vi "FlexMag - 23-03-2023.vi"() -> ()   [LabVIEW 2018] (continued)
                          n16002 = local read "abort ch2"() -> (w20214:bool)
                          n16003 = Not(x=w20216) -> (.not. x?=w20215:bool)
                          n16004 = Compound Arithmetic op=OR(w20211, w20214, w20215) -> (w20217:bool)
                        }
                      }
                      frame True {
                      }
                    }
                  }
                }
              }
              frame #6 {
                n16005 = local read "ch2 shutdown alg"() -> (w20224:bool)
                n16006 = case shown="True" w20224 {
                  frame False {
                  }
                  frame True {
                    n16007 = local read "abort ch2"() -> (w20225:bool)
                    n16008 = case shown="False" w20225 {
                      frame False {
                        n16009 = local write "ch2 sd bg bv close led"(TRUE ("ch1 sd cc close led")) -> ()
                        n16010 = Wait (ms)(milliseconds to wait=u32 1000) -> ()  [unwired: 1 out]
                      }
                      frame True {
                      }
                    }
                  }
                }
              }
              frame #7 {
                # "TP stop"
                n16011 = local read "ch2 shutdown alg"() -> (w20228:bool)
                n16012 = case shown="True" w20228 {
                  frame False {
                  }
                  frame True {
                    n16013 = local read "abort ch2"() -> (w20229:bool)
                    n16014 = case shown="False" w20229 {
                      frame False {
                        n16015 = stacked-sequence {
                          frame #0 {
                            n16016 = flat-sequence {
                              frame #0 {
                                n16017 = local write "Tp2 auto stop"(TRUE ("Tp1 auto stop")) -> ()
                                n16018 = Wait (ms)(milliseconds to wait=u32 100) -> ()  [unwired: 1 out]
                              }
                              frame #1 {
                                n16019 = Wait (ms)(milliseconds to wait=u32 5000) -> ()  [unwired: 1 out]
                              }
                              frame #2 {
                                n16020 = local write "Tp2 auto stop"(TRUE ("Tp1 auto stop")) -> ()
                                n16021 = Wait (ms)(milliseconds to wait=u32 100) -> ()  [unwired: 1 out]
                              }
                            }
                          }
                          frame #1 {
                            n16022 = while {
                              i -> [w20246]
                              stop <- w20241 stop-if-true
                              n16023 = Multiply(x=3000 ("y"), y=5) -> (x*y=w20235:i32)
                              n16024 = Greater Or Equal?(x=w20246, y=w20235) -> (x >= y?=w20240:bool)
                              n16025 = case shown="True" w20240 {
                                frame False {
                                }
                                frame True {
                                n16026 = local write "Warning Message"("CH2 ShutDown process  is canceled !\nCH2 TP couldn't be stopped" ("Warning Message")) -> ()
                                n16027 = local write "ch2 shutdown error"(TRUE ("ch1 pumpdown error")) -> ()
                                }
                              }
                              n16028 = local read "ch2 shutdown alg"() -> (w20244:bool)
                              n16029 = local read "ch2_tp_gui"() -> (w20239:bool)
                              n16030 = local read "abort ch2"() -> (w20242:bool)
                              n16031 = Not(x=w20239) -> (.not. x?=w20238:bool)
                              n16032 = Not(x=w20244) -> (.not. x?=w20243:bool)
                              n16033 = Wait Until Next ms Multiple(millisecond multiple=u32 200) -> ()  [unwired: 1 out]
                              n16034 = Compound Arithmetic op=OR(w20238, w20242, w20243) -> (w20241:bool)
                            }
                          }
                        }
                      }
                      frame True {
                      }
                    }
                  }
                }
              }
              frame #8 {
                n16035 = local read "ch2 shutdown alg"() -> (w20249:bool)
                n16036 = case shown="True" w20249 {
                  frame False {
                  }
                  frame True {
                    n16037 = local read "abort ch2"() -> (w20250:bool)
                    n16038 = case shown="False" w20250 {
                      frame False {
                        n16039 = local write "ch2 sd tp stop led"(TRUE ("ch1 sd cc close led")) -> ()
                        n16040 = Wait (ms)(milliseconds to wait=u32 1000) -> ()  [unwired: 1 out]
                      }
                      frame True {
                      }
                    }
                  }
                }
              }
              frame #9 {
                # "tp bv close"
                n16041 = local read "ch2 shutdown alg"() -> (w20253:bool)
                n16042 = case shown="True" w20253 {
                  frame False {
                  }
                  frame True {
                    n16043 = local read "abort ch2"() -> (w20254:bool)
                    n16044 = case shown="False" w20254 {
                      frame False {
                        n16045 = while {
                          i -> [w20259]
                          stop <- w20263 stop-if-true
                          n16046 = Greater?(x=w20259, y=100) -> (0:w20256:bool)
                          n16047 = case shown="True" w20256 {
                            frame False {
                            }
                            frame True {
                              n16048 = local write "Warning Message"("CH2 ShutDown process  is canceled !\nCH2 TP BV couldn't be closed" ("Warning Message")) -> ()
                              n16049 = local write "ch2 shutdown error"(TRUE ("ch1 pumpdown error")) -> ()
                            }
                          }
                          n16050 = local read "CH2_TP_BV_DI"() -> (w20255:bool)
                          n16051 = case shown="True" w20255 {
                            tunnel: [TRUE FALSE] -> w20257
                            frame False {
                            }
                            frame True {
                              n16052 = Wait Until Next ms Multiple(millisecond multiple=u32 200) -> ()  [unwired: 1 out]
                              n16053 = local write "CH2_TP_BV_DO"(FALSE ("CH1_CC_DO")) -> ()
                            }
                          }
                          n16054 = local read "ch2 shutdown alg"() -> (w20262:bool)
                          n16055 = local read "abort ch2"() -> (w20260:bool)
                          n16056 = Not(x=w20262) -> (.not. x?=w20261:bool)
                          n16057 = Compound Arithmetic op=OR(w20257, w20260, w20261) -> (w20263:bool)
                        }
                      }
                      frame True {
                      }
                    }
                  }
                }
              }
              frame #10 {
                n16058 = local read "ch2 shutdown alg"() -> (w20270:bool)
                n16059 = case shown="True" w20270 {
                  frame False {
                  }
                  frame True {
                    n16060 = local read "abort ch2"() -> (w20271:bool)
                    n16061 = case shown="False" w20271 {
                      frame False {
                        n16062 = local write "ch2 sd tp bv close led"(TRUE ("ch1 sd cc close led")) -> ()
                        n16063 = Wait (ms)(milliseconds to wait=u32 1000) -> ()  [unwired: 1 out]
                      }
                      frame True {
                      }
                    }
                  }
                }
              }
              frame #11 {
                # "mp stop"
                n16064 = local read "ch2 shutdown alg"() -> (w20274:bool)
                n16065 = case shown="True" w20274 {
                  frame False {
                  }
                  frame True {
                    n16066 = local read "abort ch2"() -> (w20275:bool)
                    n16067 = case shown="False" w20275 {
                      frame False {
                        n16068 = while {
                          i -> [w20280]
                          stop <- w20284 stop-if-true
                          n16069 = Greater?(x=w20280, y=100) -> (0:w20277:bool)
                          n16070 = case shown="True" w20277 {
                            frame False {
                            }
                            frame True {
                              n16071 = local write "Warning Message"("CH2 ShutDown process  is canceled !\nCH2 MP couldn't be stopped" ("Warning Message")) -> ()
                              n16072 = local write "ch2 shutdown error"(TRUE ("ch1 pumpdown error")) -> ()
                            }
                          }
                          n16073 = local read "CH2_MP_DI"() -> (w20276:bool)
                          n16074 = case shown="True" w20276 {
                            tunnel: [TRUE FALSE] -> w20278
                            frame False {
                            }
                            frame True {
                              n16075 = Wait Until Next ms Multiple(millisecond multiple=u32 200) -> ()  [unwired: 1 out]
                              n16076 = local write "CH2_MP_DO"(FALSE ("CH1_CC_DO")) -> ()
                            }
                          }
                          n16077 = local read "ch2 shutdown alg"() -> (w20283:bool)
                          n16078 = local read "abort ch2"() -> (w20281:bool)
                          n16079 = Not(x=w20283) -> (.not. x?=w20282:bool)
                          n16080 = Compound Arithmetic op=OR(w20278, w20281, w20282) -> (w20284:bool)
                        }
                      }
                      frame True {
                      }
                    }
                  }
                }
              }
              frame #12 {
                n16081 = local read "ch2 shutdown alg"() -> (w20291:bool)
                n16082 = case shown="True" w20291 {
                  frame False {
                  }
                  frame True {
                    n16083 = local read "abort ch2"() -> (w20292:bool)
                    n16084 = case shown="False" w20292 {
                      frame False {
                        n16085 = local write "ch2 sd mp stop led"(TRUE ("ch1 sd cc close led")) -> ()
                        n16086 = Wait (ms)(milliseconds to wait=u32 1000) -> ()  [unwired: 1 out]
                      }
                      frame True {
                      }
                    }
                  }
                }
              }
              frame #13 {
                # "pl vbv open"
                n16087 = local read "ch2 shutdown alg"() -> (w20295:bool)
                n16088 = case shown="True" w20295 {
                  frame False {
                  }
                  frame True {
                    n16089 = local read "abort ch2"() -> (w20296:bool)
                    n16090 = case shown="False" w20296 {
                      frame False {
                        n16091 = while {
                          i -> [w20301]
                          stop <- w20305 stop-if-true
                          n16092 = Greater?(x=w20301, y=100) -> (0:w20298:bool)
                          n16093 = case shown="True" w20298 {
                            frame False {
                            }
                            frame True {
                              n16094 = local write "Warning Message"("CH2 ShutDown process  is canceled !\nCH2 PL VBV couldn't be opened" ("Warning Message")) -> ()
                              n16095 = local write "ch2 shutdown error"(TRUE ("ch1 pumpdown error")) -> ()
                            }
                          }
                          n16096 = local read "CH2_PL_VBV_DI"() -> (w20297:bool)
                          n16097 = case shown="False" w20297 {
                            tunnel: [FALSE TRUE] -> w20299
                            frame False {
                              n16098 = Wait Until Next ms Multiple(millisecond multiple=u32 200) -> ()  [unwired: 1 out]
                              n16099 = local write "CH2_PL_VBV_DO"(TRUE ("CH1_CC_DO")) -> ()
                            }
                            frame True {
                            }
                          }
                          n16100 = local read "ch2 shutdown alg"() -> (w20304:bool)
                          n16101 = local read "abort ch2"() -> (w20302:bool)
                          n16102 = Not(x=w20304) -> (.not. x?=w20303:bool)
                          n16103 = Compound Arithmetic op=OR(w20299, w20302, w20303) -> (w20305:bool)
                        }
                      }
                      frame True {
                      }
                    }
                  }
                }
              }
              frame #14 {
                n16104 = local read "ch2 shutdown alg"() -> (w20312:bool)
                n16105 = case shown="True" w20312 {
                  frame False {
                  }
                  frame True {
                    n16106 = local read "abort ch2"() -> (w20313:bool)
                    n16107 = case shown="False" w20313 {
                      frame False {
                        n16108 = local write "ch2 sd pl vbv open led"(TRUE ("ch1 sd cc close led")) -> ()
                        n16109 = Wait (ms)(milliseconds to wait=u32 1000) -> ()  [unwired: 1 out]
                      }
                      frame True {
                      }
                    }
                  }
                }
              }
              frame #15 {
                n16110 = local read "ch2 shutdown alg"() -> (w20316:bool)
                n16111 = case shown="True" w20316 {
                  frame False {
                  }
                  frame True {
                    n16112 = local read "abort ch2"() -> (w20317:bool)
                    n16113 = case shown="False" w20317 {
                      frame False {
                        n16114 = local read "ch2 vent?"() -> (w20318:bool)
                        n16115 = case shown="True" w20318 {
                          frame False {
                            n16116 = stacked-sequence {
                              frame #0 {
                                n16117 = local read "ch2 shutdown alg"() -> (w20319:bool)
                                n16118 = case shown="True" w20319 {
                                frame False {
                                }
                                frame True {
                                n16119 = flat-sequence {
                                frame #0 {
                                n16120 = local write "pcgv2 auto close"(TRUE ("pcgv1 auto open")) -> ()
                                }
                                frame #1 {
                                n16121 = Wait (ms)(milliseconds to wait=u32 2000) -> ()  [unwired: 1 out]
                                }
                                frame #2 {
                                n16122 = local write "pcgv2 auto close"(TRUE ("pcgv1 auto open")) -> ()
                                }
                                }
                                }
                                }
                              }
                              frame #1 {
                                n16123 = while {
                                i -> [w20330]
                                stop <- w20326 stop-if-true
                                n16124 = Greater Or Equal?(x=w20330, y=200) -> (x >= y?=w20332:bool)
                                n16125 = case shown="True" w20332 {
                                frame False {
                                }
                                frame True {
                                n16126 = local write "ch2 shutdown error"(TRUE ("ch1 pumpdown error")) -> ()
                                n16127 = local write "Warning Message"("CH2 ShutDown process  is canceled !\nCH2 PC GV couldn't be closed" ("Warning Message")) -> ()
                                }
                                }
                                n16128 = local read "ch2_pcgv_gui"() -> (w20323:bool)
                                n16129 = local read "abort ch2"() -> (w20327:bool)
                                n16130 = local read "ch2 shutdown alg"() -> (w20329:bool)
                                n16131 = Wait Until Next ms Multiple(millisecond multiple=u32 200) -> ()  [unwired: 1 out]
                                n16132 = Not(x=w20323) -> (.not. x?=w20324:bool)
                                n16133 = Not(x=w20329) -> (.not. x?=w20328:bool)
                                n16134 = Compound Arithmetic op=OR(w20324, w20327, w20328) -> (w20326:bool)
                                }
                              }
                            }
                          }
                          frame True {
                            n16135 = stacked-sequence {
                              frame #0 {
                                n16136 = local read "ch2 shutdown alg"() -> (w20335:bool)
                                n16137 = case shown="True" w20335 {
                                frame False {
                                }
                                frame True {
                                n16138 = flat-sequence {
                                frame #0 {
                                n16139 = local write "pcgv2 auto open"(TRUE ("pcgv1 auto open")) -> ()
                                }
                                frame #1 {
                                n16140 = Wait (ms)(milliseconds to wait=u32 2000) -> ()  [unwired: 1 out]
                                }
                                frame #2 {
                                n16141 = local write "pcgv2 auto open"(TRUE ("pcgv1 auto open")) -> ()
                                }
                                }
                                }
                                }
                              }
                              frame #1 {
                                n16142 = while {
                                i -> [w20345]
                                stop <- w20341 stop-if-true
                                n16143 = Greater Or Equal?(x=w20345, y=200) -> (x >= y?=w20347:bool)
                                n16144 = case shown="True" w20347 {
                                frame False {
                                }
                                frame True {
                                n16145 = local write "ch2 shutdown error"(TRUE ("ch1 pumpdown error")) -> ()
                                n16146 = local write "Warning Message"("CH2 ShutDown process  is canceled !\nCH2 PC GV couldn't be opened" ("Warning Message")) -> ()
                                }
                                }
                                n16147 = local read "ch2 shutdown alg"() -> (w20344:bool)
                                n16148 = local read "ch2_pcgv_gui"() -> (w20340:bool)
                                n16149 = local read "abort ch2"() -> (w20342:bool)
                                n16150 = Wait Until Next ms Multiple(millisecond multiple=u32 200) -> ()  [unwired: 1 out]
                                n16151 = Not(x=w20344) -> (.not. x?=w20343:bool)
                                n16152 = Compound Arithmetic op=OR(w20340, w20342, w20343) -> (w20341:bool)
                                }
                              }
                            }
                          }
                        }
                      }
                      frame True {
                      }
                    }
                  }
                }
              }
              frame #16 {
                n16153 = local read "ch2 shutdown alg"() -> (w20350:bool)
                n16154 = case shown="True" w20350 {
                  frame False {
                  }
                  frame True {
                    n16155 = local read "abort ch2"() -> (w20351:bool)
                    n16156 = case shown="False" w20351 {
                      frame False {
                        n16157 = local read "ch2 vent?"() -> (w20352:bool)
                        n16158 = case shown="True" w20352 {
                          frame False {
                            n16159 = local write "ch2 sd pcgv close led"(TRUE ("ch1 sd cc close led")) -> ()
                            n16160 = Wait (ms)(milliseconds to wait=u32 1000) -> ()  [unwired: 1 out]
                          }
                          frame True {
                            n16161 = local write "ch2 sd pcgv open led"(TRUE ("ch1 sd cc close led")) -> ()
                            n16162 = Wait (ms)(milliseconds to wait=u32 1000) -> ()  [unwired: 1 out]
                          }
                        }
                      }
                      frame True {
                      }
                    }
                  }
                }
              }
              frame #17 {
                n16163 = local read "ch2 shutdown alg"() -> (w20357:bool)
                n16164 = case shown="True" w20357 {
                  frame False {
                  }
                  frame True {
                    n16165 = local read "abort ch2"() -> (w20358:bool)
                    n16166 = case shown="False" w20358 {
                      frame False {
                        n16167 = local read "ch2 vent?"() -> (w20359:bool)
                        n16168 = case shown="True" w20359 {
                          frame False {
                            n16169 = while {
                              i -> [w20366]
                              stop <- w20362 stop-if-true
                              n16170 = Greater Or Equal?(x=w20366, y=200) -> (x >= y?=w20368:bool)
                              n16171 = case shown="True" w20368 {
                                frame False {
                                }
                                frame True {
                                n16172 = local write "ch2 shutdown error"(TRUE ("ch1 pumpdown error")) -> ()
                                n16173 = local write "Warning Message"("CH2 ShutDown process  is canceled !\nCH2 Trns BP Left couldn't be closed" ("Warning Message")) -> ()
                                }
                              }
                              n16174 = local read "CH2_Trns_BP_Left_DI"() -> (w20361:bool)
                              n16175 = case shown="True" w20361 {
                                tunnel: [TRUE FALSE] -> w20360
                                frame False {
                                }
                                frame True {
                                n16176 = Wait Until Next ms Multiple(millisecond multiple=u32 200) -> ()  [unwired: 1 out]
                                n16177 = local write "CH2_Trns_BP_Left_DO"(FALSE ("CH1_WFC_DO")) -> ()
                                }
                              }
                              n16178 = local read "abort ch2"() -> (w20363:bool)
                              n16179 = local read "ch2 shutdown alg"() -> (w20365:bool)
                              n16180 = Not(x=w20365) -> (.not. x?=w20364:bool)
                              n16181 = Compound Arithmetic op=OR(w20360, w20363, w20364) -> (w20362:bool)
                            }
                          }
                          frame True {
                            n16182 = local read "ch2_3 vacuum level"() -> (w20375:string)
                            n16183 = Equal?(x=w20375, y="VACUUM") -> (x = y?=w20376:bool)
                            n16184 = case shown="True" w20376 {
                              frame False {
                              }
                              frame True {
                                n16185 = while {
                                i -> [w20384]
                                stop <- w20380 stop-if-true
                                n16186 = Greater Or Equal?(x=w20384, y=100) -> (x >= y?=w20386:bool)
                                n16187 = case shown="True" w20386 {
                                frame False {
                                }
                                frame True {
                                n16188 = local write "ch2 shutdown error"(TRUE ("ch1 pumpdown error")) -> ()
                                n16189 = local write "Warning Message"("CH2 ShutDown process  is canceled !\nCH2 Trns BP Left couldn't be opened" ("Warning Message")) -> ()
                                }
                                }
                                n16190 = local read "CH2_Trns_BP_Left_DI"() -> (w20379:bool)
                                n16191 = case shown="False" w20379 {
                                tunnel: [FALSE TRUE] -> w20378
                                frame False {
                                n16192 = Wait Until Next ms Multiple(millisecond multiple=u32 200) -> ()  [unwired: 1 out]
                                n16193 = local write "CH2_Trns_BP_Left_DO"(TRUE ("CH1_WFC_DO")) -> ()
                                }
                                frame True {
                                }
                                }
                                n16194 = local read "ch2 shutdown alg"() -> (w20383:bool)
                                n16195 = local read "abort ch2"() -> (w20381:bool)
                                n16196 = Not(x=w20383) -> (.not. x?=w20382:bool)
                                n16197 = Compound Arithmetic op=OR(w20378, w20381, w20382) -> (w20380:bool)
                                }
                              }
                            }
                          }
                        }
                      }
                      frame True {
                      }
                    }
                  }
                }
              }
              frame #18 {
                n16198 = local read "ch2 shutdown alg"() -> (w20393:bool)
                n16199 = case shown="True" w20393 {
                  frame False {
                  }
                  frame True {
                    n16200 = local read "abort ch2"() -> (w20394:bool)
                    n16201 = case shown="False" w20394 {
                      frame False {
                        n16202 = local read "ch2 vent?"() -> (w20395:bool)
                        n16203 = case shown="False" w20395 {
                          frame False {
                            n16204 = local write "ch2 sd trns bp left close led"(TRUE ("ch1 sd cc close led")) -> ()
                            n16205 = Wait (ms)(milliseconds to wait=u32 1000) -> ()  [unwired: 1 out]
                          }
                          frame True {
                            n16206 = local write "ch2 sd trns bp left open led"(TRUE ("ch1 sd cc close led")) -> ()
                            n16207 = Wait (ms)(milliseconds to wait=u32 1000) -> ()  [unwired: 1 out]
                          }
                        }
                      }
                      frame True {
                      }
                    }
                  }
                }
              }
              frame #19 {
                n16208 = local read "ch2 shutdown alg"() -> (w20400:bool)
                n16209 = case shown="True" w20400 {
                  frame False {
                  }
                  frame True {
                    n16210 = local read "abort ch2"() -> (w20401:bool)
                    n16211 = case shown="False" w20401 {
                      frame False {
                        n16212 = local read "ch2 vent?"() -> (w20402:bool)
                        n16213 = case shown="True" w20402 {
                          frame False {
                            n16214 = while {
                              i -> [w20409]
                              stop <- w20405 stop-if-true
                              n16215 = Greater Or Equal?(x=w20409, y=200) -> (x >= y?=w20411:bool)
                              n16216 = case shown="True" w20411 {
                                frame False {
                                }
                                frame True {
                                n16217 = local write "ch2 shutdown error"(TRUE ("ch1 pumpdown error")) -> ()
                                n16218 = local write "Warning Message"("CH2 ShutDown process  is canceled !\nCH2 Trns BP Right couldn't be closed" ("Warning Message")) -> ()
                                }
                              }
                              n16219 = local read "CH2_Trns_BP_Right_DI"() -> (w20404:bool)
                              n16220 = case shown="True" w20404 {
                                tunnel: [TRUE FALSE] -> w20403
                                frame False {
                                }
                                frame True {
                                n16221 = Wait Until Next ms Multiple(millisecond multiple=u32 200) -> ()  [unwired: 1 out]
                                n16222 = local write "CH2_Trns_BP_Right_DO"(FALSE ("CH1_WFC_DO")) -> ()
                                }
                              }
                              n16223 = local read "abort ch2"() -> (w20406:bool)
                              n16224 = local read "ch2 shutdown alg"() -> (w20408:bool)
                              n16225 = Not(x=w20408) -> (.not. x?=w20407:bool)
                              n16226 = Compound Arithmetic op=OR(w20403, w20406, w20407) -> (w20405:bool)
                            }
                          }
                          frame True {
                            n16227 = local read "ch1_2 vacuum level"() -> (w20419:string)
                            n16228 = Equal?(x=w20419, y="VACUUM") -> (x = y?=w20418:bool)
                            n16229 = case shown="True" w20418 {
                              frame False {
                              }
                              frame True {
                                n16230 = while {
                                i -> [w20427]
                                stop <- w20423 stop-if-true
                                n16231 = Greater Or Equal?(x=w20427, y=100) -> (x >= y?=w20429:bool)
                                n16232 = case shown="True" w20429 {
                                frame False {
                                }
                                frame True {
                                n16233 = local write "ch2 shutdown error"(TRUE ("ch1 pumpdown error")) -> ()
                                n16234 = local write "Warning Message"("CH2 ShutDown process  is canceled !\nCH2 Trns BP Right couldn't be opened" ("Warning Message")) -> ()
                                }
                                }
                                n16235 = local read "CH2_Trns_BP_Right_DI"() -> (w20422:bool)
                                n16236 = case shown="False" w20422 {
                                tunnel: [FALSE TRUE] -> w20421
                                frame False {
                                n16237 = Wait Until Next ms Multiple(millisecond multiple=u32 200) -> ()  [unwired: 1 out]
                                n16238 = local write "CH2_Trns_BP_Right_DO"(TRUE ("CH1_WFC_DO")) -> ()
                                }
                                frame True {
                                }
                                }
                                n16239 = local read "ch2 shutdown alg"() -> (w20426:bool)
                                n16240 = local read "abort ch2"() -> (w20424:bool)
                                n16241 = Not(x=w20426) -> (.not. x?=w20425:bool)
                                n16242 = Compound Arithmetic op=OR(w20421, w20424, w20425) -> (w20423:bool)
                                }
                              }
                            }
                          }
                        }
                      }
                      frame True {
                      }
                    }
                  }
                }
              }
              frame #20 {
                n16243 = local read "ch2 shutdown alg"() -> (w20436:bool)
                n16244 = case shown="True" w20436 {
                  frame False {
                  }
                  frame True {
                    n16245 = local read "abort ch2"() -> (w20437:bool)
                    n16246 = case shown="False" w20437 {
                      frame False {
                        n16247 = local read "ch2 vent?"() -> (w20438:bool)
                        n16248 = case shown="False" w20438 {
                          frame False {
                            n16249 = local write "ch2 sd trns bp right close led"(TRUE ("ch1 sd cc close led")) -> ()
                            n16250 = Wait (ms)(milliseconds to wait=u32 1000) -> ()  [unwired: 1 out]
                          }
                          frame True {
                            n16251 = local write "ch2 sd trns bp right open led"(TRUE ("ch1 sd cc close led")) -> ()
                            n16252 = Wait (ms)(milliseconds to wait=u32 1000) -> ()  [unwired: 1 out]
                          }
                        }
                      }
                      frame True {
                      }
                    }
                  }
                }
              }
              frame #21 {
                n16253 = local read "ch2 shutdown alg"() -> (w20443:bool)
                n16254 = case shown="True" w20443 {
                  frame False {
                  }
                  frame True {
                    n16255 = local read "abort ch2"() -> (w20444:bool)
                    n16256 = case shown="False" w20444 {
                      frame False {
                        n16257 = local read "ch2 vent?"() -> (w20445:bool)
                        n16258 = case shown="True" w20445 {
                          frame False {
                          }
                          frame True {
                            n16259 = while {
                              i -> [w20448]
                              stop <- w20451 stop-if-true
                              n16260 = Greater?(x=w20448, y=100) -> (0:w20447:bool)
                              n16261 = case shown="True" w20447 {
                                frame False {
                                }
                                frame True {
                                n16262 = local write "Warning Message"("CH2 ShutDown process  is canceled !\nCH2 CH VBV couldn't be opened" ("Warning Message")) -> ()
                                n16263 = local write "ch2 shutdown error"(TRUE ("ch1 pumpdown error")) -> ()
                                }
                              }
                              n16264 = local read "CH2_CH_VBV_DI"() -> (w20446:bool)
                              n16265 = case shown="False" w20446 {
                                tunnel: [FALSE TRUE] -> w20450
                                frame False {
                                n16266 = Wait Until Next ms Multiple(millisecond multiple=u32 200) -> ()  [unwired: 1 out]
                                n16267 = local write "CH2_CH_VBV_DO"(TRUE ("CH1_WFC_DO")) -> ()
                                }
                                frame True {
                                }
                              }
                              n16268 = local read "ch2 shutdown alg"() -> (w20452:bool)
                              n16269 = local read "abort ch2"() -> (w20454:bool)
                              n16270 = Not(x=w20452) -> (.not. x?=w20453:bool)
                              n16271 = Compound Arithmetic op=OR(w20450, w20454, w20453) -> (w20451:bool)
                            }
                          }
                        }
                      }
                      frame True {
                      }
                    }
                  }
                }
              }
              frame #22 {
                n16272 = local read "ch2 shutdown alg"() -> (w20461:bool)
                n16273 = case shown="True" w20461 {
                  frame False {
                  }
                  frame True {
                    n16274 = local read "abort ch2"() -> (w20462:bool)
                    n16275 = case shown="False" w20462 {
                      frame False {
                        n16276 = local read "ch2 vent?"() -> (w20463:bool)
                        n16277 = case shown="True" w20463 {
                          frame False {
                          }
                          frame True {
                            n16278 = local write "ch2 sd ch vbv open led"(TRUE ("ch1 sd cc close led")) -> ()
                            n16279 = Wait (ms)(milliseconds to wait=u32 1000) -> ()  [unwired: 1 out]
                          }
                        }
                      }
                      frame True {
                      }
                    }
                  }
                }
              }
              frame #23 {
                n16280 = local read "ch2 shutdown alg"() -> (w20466:bool)
                n16281 = case shown="True" w20466 {
                  frame False {
                  }
                  frame True {
                    n16282 = local read "abort ch2"() -> (w20467:bool)
                    n16283 = case shown="False" w20467 {
                      frame False {
                        n16284 = local read "ch2 vent?"() -> (w20468:bool)
                        n16285 = case shown="True" w20468 {
                          frame False {
                            n16286 = while {
                              i -> [w20475]
                              stop <- w20471 stop-if-true
                              # "10min"
                              n16287 = Greater Or Equal?(x=w20475, y=3000) -> (x >= y?=w20477:bool)
                              n16288 = case shown="True" w20477 {
                                frame False {
                                }
                                frame True {
                                n16289 = local write "ch2 shutdown error"(TRUE ("ch1 pumpdown error")) -> ()
                                n16290 = local write "Warning Message"("CH2 ShutDown process  is canceled !\nCH2 PL ATM switch  couldn't be opened" ("Warning Message")) -> ()
                                }
                              }
                              n16291 = local read "CH2_PL_ATM_DI"() -> (w20469:bool)
                              n16292 = local read "abort ch2"() -> (w20472:bool)
                              n16293 = local read "ch2 shutdown alg"() -> (w20474:bool)
                              n16294 = case shown="False" w20469 {
                                tunnel: [FALSE TRUE] -> w20470
                                frame False {
                                n16295 = Wait Until Next ms Multiple(millisecond multiple=u32 200) -> ()  [unwired: 1 out]
                                }
                                frame True {
                                }
                              }
                              n16296 = Not(x=w20474) -> (.not. x?=w20473:bool)
                              n16297 = Compound Arithmetic op=OR(w20470, w20472, w20473) -> (w20471:bool)
                            }
                          }
                          frame True {
                            n16298 = while {
                              i -> [w20491]
                              stop <- w20487 stop-if-true
                              # "10min"
                              n16299 = Greater Or Equal?(x=w20491, y=3000) -> (x >= y?=w20493:bool)
                              n16300 = case shown="True" w20493 {
                                frame False {
                                }
                                frame True {
                                n16301 = local write "ch2 shutdown error"(TRUE ("ch1 pumpdown error")) -> ()
                                n16302 = local write "Warning Message"("CH2 ShutDown process  is canceled !\nCH2 ATM switches  couldn't be opened" ("Warning Message")) -> ()
                                }
                              }
                              n16303 = local read "CH2_CH_ATM_DI"() -> (w20485:bool)
                              n16304 = local read "CH2_PL_ATM_DI"() -> (w20484:bool)
                              n16305 = And(x=w20485, y=w20484) -> (x .and. y?=w20483:bool)
                              n16306 = local read "abort ch2"() -> (w20488:bool)
                              n16307 = local read "ch2 shutdown alg"() -> (w20490:bool)
                              n16308 = case shown="False" w20483 {
                                tunnel: [FALSE TRUE] -> w20486
                                frame False {
                                n16309 = Wait Until Next ms Multiple(millisecond multiple=u32 200) -> ()  [unwired: 1 out]
                                }
                                frame True {
                                }
                              }
                              n16310 = Not(x=w20490) -> (.not. x?=w20489:bool)
                              n16311 = Compound Arithmetic op=OR(w20486, w20488, w20489) -> (w20487:bool)
                            }
                          }
                        }
                      }
                      frame True {
                      }
                    }
                  }
                }
              }
              frame #24 {
                n16312 = local read "ch2 shutdown alg"() -> (w20499:bool)
                n16313 = case shown="True" w20499 {
                  frame False {
                  }
                  frame True {
                    n16314 = local read "abort ch2"() -> (w20500:bool)
                    n16315 = case shown="False" w20500 {
                      frame False {
                        n16316 = local read "ch2 vent?"() -> (w20501:bool)
                        n16317 = case shown="True" w20501 {
                          frame False {
                            n16318 = local write "ch2 sd PL atm on led"(TRUE ("ch1 sd cc close led")) -> ()
                            n16319 = Wait (ms)(milliseconds to wait=u32 1000) -> ()  [unwired: 1 out]
                          }
                          frame True {
                            w20505 = FALSE ("ch1 sd cc close led")
                            w20506 = "ATMOSPHERE" ("ch3_4 vacuum level")
                            n16320 = local write "CH2_Trns_BP_Right_DO"(w20505) -> ()
                            n16321 = local write "CH2_Trns_BP_Left_DO"(w20505) -> ()
                            n16322 = local write "pcgv2 auto close"(TRUE ("pcgv2 auto close")) -> ()
                            n16323 = Wait (ms)(milliseconds to wait=u32 500) -> ()  [unwired: 1 out]
                            n16324 = local write "ch2 sd PL-CH atm on led"(TRUE ("ch1 sd cc close led")) -> ()
                            n16325 = local write "ch1_2 vacuum level"(w20506) -> ()
                            n16326 = local write "ch2_3 vacuum level"(w20506) -> ()
                          }
                        }
                      }
                      frame True {
                      }
                    }
                  }
                }
              }
              frame #25 {
                n16327 = local read "ch2 shutdown alg"() -> (w20509:bool)
                n16328 = case shown="True" w20509 {
                  frame False {
                  }
                  frame True {
                    n16329 = local read "abort ch2"() -> (w20510:bool)
                    n16330 = case shown="False" w20510 {
                      frame False {
                        n16331 = local read "ch2 vent?"() -> (w20511:bool)
                        n16332 = case shown="False" w20511 {
                          frame False {
                            w20514 = TRUE ("Buzzer DO")
                            n16333 = local write "Buzzer DO"(w20514) -> ()
                            n16334 = local write "ch2 sd completed led"(w20514) -> ()
                            n16335 = Wait (ms)(milliseconds to wait=u32 3000) -> ()  [unwired: 1 out]
                            n16336 = local write "System Status"("CH2 SHUTDOWN PROCESS COMPLETED" ("System Status")) -> ()
                          }
                          frame True {
                            w20515 = TRUE ("Buzzer DO")
                            n16337 = local write "Buzzer DO"(w20515) -> ()
                            n16338 = local write "ch2 sd completed led"(w20515) -> ()
                            n16339 = Wait (ms)(milliseconds to wait=u32 3000) -> ()  [unwired: 1 out]
                            n16340 = local write "System Status"("CH2 VENT PROCESS COMPLETED" ("System Status")) -> ()
                          }
                        }
                      }
                      frame True {
                      }
                    }
                  }
                }
              }
              frame #26 {
                n16341 = local read "ch2 shutdown alg"() -> (w20518:bool)
                n16342 = case shown="True" w20518 {
                  frame False {
                  }
                  frame True {
                    n16343 = local read "abort ch2"() -> (w20519:bool)
                    n16344 = case shown="False" w20519 {
                      frame False {
                        w20521 = FALSE ("Buzzer DO")
                        n16345 = local write "Buzzer DO"(w20521) -> ()
                        n16346 = local write "ch2 shutdown alg"(w20521) -> ()
                        n16347 = local write "Shut Down CH2"(w20521) -> ()
                        n16348 = Wait (ms)(milliseconds to wait=u32 3000) -> ()  [unwired: 1 out]
                        n16349 = local write "System Status"("SEMI-AUTOMATIC MODE " ("System Status")) -> ()
                      }
                      frame True {
                      }
                    }
                  }
                }
              }
            }
          }
          frame True {
          }
        }
      }
    }
  }
  n16350 = while {
    stop <- FALSE stop-if-true
    n16351 = Wait Until Next ms Multiple(millisecond multiple=u32 300) -> ()  [unwired: 1 out]
    n16352 = case shown="True" "ch3 pumpdown alg" {
      frame False {
      }
      frame True {
        n16353 = local read "abort ch3"() -> (w21448:bool)
        n16354 = case shown="False" w21448 {
          frame False {
            n16355 = stacked-sequence {
              frame #0 {
                n16356 = stacked-sequence {
                  frame #0 {
                    n16357 = local write "ch3 pd clear"(TRUE ("ch1 pd clear")) -> ()
                    n16358 = Wait (ms)(milliseconds to wait=u32 100) -> ()  [unwired: 1 out]
                  }
                  frame #1 {
                    n16359 = local write "System Status"("CH3 PUMPDOWN PROCESS IN PROGRESS" ("System Status")) -> ()
                  }
                  frame #2 {
                    n16360 = local read "CH3_DS_DI"() -> (w21452:bool)
                    n16361 = case shown="False" w21452 {
                      frame False {
                        n16362 = stacked-sequence {
                          frame #0 {
                            n16363 = local write "Buzzer DO"(TRUE ("Buzzer DO")) -> ()
                            n16364 = Wait (ms)(milliseconds to wait=u32 100) -> ()  [unwired: 1 out]
                          }
                          frame #1 {
                            n16365 = while {
                              i -> [w21457]
                              stop <- w21460 stop-if-true
                              n16366 = Greater?(x=w21457, y=900) -> (0:w21456:bool)
                              n16367 = case shown="True" w21456 {
                                frame False {
                                }
                                frame True {
                                n16368 = local write "Warning Message"("CH3 PumpDown process  is canceled !\nCH3 Door is open" ("Warning Message")) -> ()
                                n16369 = local write "ch3 pumpdown error"(TRUE ("ch1 pumpdown error")) -> ()
                                }
                              }
                              n16370 = local read "CH3_DS_DI"() -> (w21455:bool)
                              n16371 = case shown="True" w21455 {
                                tunnel: [FALSE TRUE] -> w21459
                                frame False {
                                n16372 = Wait Until Next ms Multiple(millisecond multiple=u32 200) -> ()  [unwired: 1 out]
                                }
                                frame True {
                                n16373 = local write "Buzzer DO"(FALSE ("Buzzer DO")) -> ()
                                }
                              }
                              n16374 = local read "ch3 pumpdown alg"() -> (w21461:bool)
                              n16375 = local read "abort ch3"() -> (w21463:bool)
                              n16376 = Not(x=w21461) -> (.not. x?=w21462:bool)
                              n16377 = Compound Arithmetic op=OR(w21459, w21463, w21462) -> (w21460:bool)
                            }
                          }
                        }
                      }
                      frame True {
                      }
                    }
                  }
                  frame #3 {
                    n16378 = disable-structure shown="Disabled" {
                      frame Disabled {
                        n16379 = while {
                          i -> [w21472]
                          stop <- w21475 stop-if-true
                          n16380 = Greater?(x=w21472, y=900) -> (0:w21471:bool)
                          n16381 = case shown="True" w21471 {
                            frame False {
                            }
                            frame True {
                              n16382 = local write "Warning Message"("CH3 PumpDown process  is canceled !\nCH3 Water Switch couldn't be opened" ("Warning Message")) -> ()
                              n16383 = local write "ch3 pumpdown error"(TRUE ("ch1 pumpdown error")) -> ()
                            }
                          }
                          n16384 = local read "CH3_WFC_DI"() -> (w21470:bool)
                          n16385 = case shown="False" w21470 {
                            tunnel: [FALSE TRUE] -> w21474
                            frame False {
                              n16386 = Wait Until Next ms Multiple(millisecond multiple=u32 200) -> ()  [unwired: 1 out]
                              n16387 = local write "CH3_WFC_DO"(TRUE ("CH1_WFC_DO")) -> ()
                            }
                            frame True {
                            }
                          }
                          n16388 = local read "ch3 pumpdown alg"() -> (w21476:bool)
                          n16389 = local read "abort ch3"() -> (w21478:bool)
                          n16390 = Not(x=w21476) -> (.not. x?=w21477:bool)
                          n16391 = Compound Arithmetic op=OR(w21474, w21478, w21477) -> (w21475:bool)
                        }
                      }
                      frame Enabled {
                      }
                    }
                  }
                }
              }
              frame #1 {
                # "ATM switches close"
                n16392 = local read "ch3 pumpdown alg"() -> (w21485:bool)
                n16393 = case shown="True" w21485 {
                  frame False {
                  }
                  frame True {
                    n16394 = local read "abort ch3"() -> (w21486:bool)
                    n16395 = case shown="False" w21486 {
                      frame False {
                        w21488 = FALSE ("CH1_PL_ATM_DO")
                        n16396 = local write "CH3_PL_ATM_DO"(w21488) -> ()
                        n16397 = local write "CH3_CH_ATM_DO"(w21488) -> ()
                        n16398 = Wait (ms)(milliseconds to wait=u32 3000) -> ()  [unwired: 1 out]
                      }
                      frame True {
                      }
                    }
                  }
                }
              }
              frame #2 {
                n16399 = local read "ch3 pumpdown alg"() -> (w21489:bool)
                n16400 = case shown="True" w21489 {
                  frame False {
                  }
                  frame True {
                    n16401 = local read "abort ch3"() -> (w21490:bool)
                    n16402 = case shown="False" w21490 {
                      frame False {
                        n16403 = local write "ch3 atms close led"(TRUE ("CH1_PL_ATM_DO")) -> ()
                        n16404 = Wait (ms)(milliseconds to wait=u32 1000) -> ()  [unwired: 1 out]
                      }
                      frame True {
                      }
                    }
                  }
                }
              }
              frame #3 {
                # "ch vbv close"
                n16405 = local read "ch3 pumpdown alg"() -> (w21493:bool)
                n16406 = case shown="True" w21493 {
                  frame False {
                  }
                  frame True {
                    n16407 = local read "abort ch3"() -> (w21494:bool)
                    n16408 = case shown="False" w21494 {
                      frame False {
                        n16409 = while {
                          i -> [w21497]
                          stop <- w21500 stop-if-true
                          n16410 = Greater Or Equal?(x=w21497, y=100) -> (x >= y?=w21498:bool)
                          n16411 = case shown="True" w21498 {
                            frame False {
                            }
                            frame True {
                              n16412 = local write "Warning Message"("CH3 PumpDown process  is canceled !\nCH3 CH VBV couldn't be closed" ("Warning Message")) -> ()
                              n16413 = local write "ch3 pumpdown error"(TRUE ("ch1 pumpdown error")) -> ()
                            }
                          }
                          n16414 = local read "CH3_CH_VBV_DI"() -> (w21495:bool)
                          n16415 = local read "ch3 pumpdown alg"() -> (w21503:bool)
                          n16416 = case shown="True" w21495 {
                            tunnel: [TRUE FALSE] -> w21499
                            frame False {
                            }
                            frame True {
                              n16417 = local write "CH3_CH_VBV_DO"(FALSE ("CH1_CH_VBV_DO")) -> ()
                              n16418 = Wait Until Next ms Multiple(millisecond multiple=u32 200) -> ()  [unwired: 1 out]
                            }
                          }
                          n16419 = local read "abort ch3"() -> (w21501:bool)
                          n16420 = Not(x=w21503) -> (.not. x?=w21502:bool)
                          n16421 = Compound Arithmetic op=OR(w21499, w21501, w21502) -> (w21500:bool)
                        }
                      }
                      frame True {
                      }
                    }
                  }
                }
              }
              frame #4 {
                n16422 = local read "ch3 pumpdown alg"() -> (w21510:bool)
                n16423 = case shown="True" w21510 {
                  frame False {
                  }
                  frame True {
                    n16424 = local read "abort ch3"() -> (w21511:bool)
                    n16425 = case shown="False" w21511 {
                      frame False {
                        n16426 = local write "ch3 ch vbv close led"(TRUE ("ch1 ch vbv close")) -> ()
                        n16427 = Wait (ms)(milliseconds to wait=u32 1000) -> ()  [unwired: 1 out]
                      }
                      frame True {
                      }
                    }
                  }
                }
              }
              frame #5 {
                # "pl vbv close"
                n16428 = local read "ch3 pumpdown alg"() -> (w21514:bool)
                n16429 = case shown="True" w21514 {
                  frame False {
                  }
                  frame True {